vi "UHR-Fleezers Control (host) - Avogadro v2.vi"() -> ()   [LabVIEW 2014] (continued)
            }
            frame Enabled {
            }
          }
          "connection reference" <- w1502
          n930 = local write "connection reference"(w1502) -> ()
          n931 = local write "Database link"(w1501) -> ()
        }
        frame #3 {
          # "Load active calibration to fpga"
          n932 = local read "Base N trap periods"() -> (w1506:u32)
          n933 = local read "T1 Osc Enable"() -> (w1505:bool)
          n934 = property on="T1 Osc Enable" class="Bool (strict)"("Val(Sgnl)"=w1505) -> ()  [unwired: 2 in, 2 out]
          n935 = property on="Base N trap periods" class="DigNum (strict)"("Val(Sgnl)"=w1506) -> ()  [unwired: 2 in, 2 out]
        }
      }
    }
    frame #4 {
      # "Set FIFO size and run FPGA"
      n936 = local read "FPGA error out"() -> (w1508:errorcluster)
      n937 = xnode "Invoke Method"("FPGA VI Reference In"=w1509, "error in"=w1508, "Requested Depth"="Trap AI FIFO Depth") -> ("FPGA VI Reference Out"=w1513:T40, "error out"=w1514:errorcluster)  [unwired: 1 out]
      n938 = xnode "Invoke Method"("FPGA VI Reference In"=w1513, "error in"=w1514, "Requested Depth"="Trap Position FIFO Depth") -> ("FPGA VI Reference Out"=w1511:T40, "error out"=w1510:errorcluster)  [unwired: 1 out]
      n939 = xnode "Invoke Method"("FPGA VI Reference In"=w1511, "error in"=w1510) -> ("error out"=w1507:errorcluster)  [unwired: 1 in, 1 out]
      n940 = local write "FPGA error out"(w1507) -> ()
    }
    frame #5 {
      # "Adjust FPGA timing loop phases"
      n941 = flat-sequence "Initial FPGA Loop Relative Phase Adjustment" {
        tunnel: "Initial Phase Adjustment (AI1)" -> [w1548]
        tunnel: "Initial Phase Adjustment (GI)" -> [w1547]
        tunnel: "Initial Phase Adj. (MCL)" -> [w1546]
        tunnel: [w1549] -> w1533
        tunnel: [w1545] -> w1532
        tunnel: "Initial Phase Adjustment (APD Acq)" -> [w1544]
        tunnel: "Initial Phase Adjustment (APD 1 Gate)" -> [w1543]
        tunnel: "Initial Phase Adjustment (Green FB)" -> [w1542]
        tunnel: "Initial Phase Adjustment (GI) 2" -> [w1541]
        tunnel: "Initial Phase Adjustment (APD 2 Gate)" -> [w1540]
        tunnel: "Initial Phase Adjustment (RI)" -> [w1539]
        tunnel: "Initial Phase Adjustment (BI DO)" -> [w1538]
        tunnel: "Initial Phase Adjustment (BI AO)" -> [w1537]
        tunnel: "Initial Phase Adjustment (APD 3 Gate)" -> [w1536]
        tunnel: w1518 -> [w1535]
        tunnel: w1533 -> [w1551]
        tunnel: [w1552] -> w1531
        tunnel: w1532 -> [w1552]
        tunnel: [w1551] -> w1530
        tunnel: w1531 -> [w1556]
        tunnel: w1530 -> [w1555]
        tunnel: [w1553] -> w1517
        frame #0 {
          n942 = local read "FPGA error out"() -> (w1534:errorcluster)
          n943 = xnode "Read/Write Control"("FPGA VI Reference In"=w1535, "error in"=w1534, "Phase count adjustment"=w1548, "Phase count adjustment (GI)"=w1547, "Phase count adjustment (MCL)"=w1546, "Phase Count Adjustment (APD Acq)"=w1544, "Phase count adjustment (APD 1 Gate)"=w1543, "Phase count adjustment (APD 2 Gate)"=w1540, "Phase count adjustment (Green FB)"=w1542, "Phase count adjustment (GI) 2"=w1541, "Phase count adjustment (RI)"=w1539, "Phase count adjustment (BI AO)"=w1537, "Phase count adjustment (BI D)"=w1538, "Phase count adjustment (APD 3 Gate)"=w1536) -> ("FPGA VI Reference Out"=w1545:T40, "error out"=w1549:errorcluster)
        }
        frame #1 {
          n944 = Wait (ms)(milliseconds to wait=u32 100) -> ()  [unwired: 1 out]
        }
        frame #2 {
          w1554 = TRUE
          n945 = xnode "Read/Write Control"("FPGA VI Reference In"=w1556, "error in"=w1555, "+ phase"=w1554, "+ phase (GI)"=w1554, "+ phase (MCL)"=w1554, "+ phase (APD Acq)"=w1554, "+ phase (APD 1 Gate)"=w1554, "+ phase (APD 2 Gate)"=w1554, "+ phase (Green FB)"=w1554, "+ phase (GI) 2"=w1554, "+ phase (RI)"=w1554, "+ phase (BI AO)"=w1554, "+ phase (BI D)"=w1554, "+ phase (APD 3 Gate)"=w1554) -> ("error out"=w1553:errorcluster)  [unwired: 1 out]
        }
      }
      n946 = local write "FPGA error out"(w1517) -> ()
    }
    frame #6 {
      w1572 = 6.0  # clock mult.
      w1571 = 49152000.0  # TCXO frequ.
      w1576 = 6.0  # clock mult.
      w1577 = 49152000.0  # TCXO frequ.
      # "Added by ronen - definition of \nlimit frequencies when using dynamic feedback"
      # "Initialize trap RF synth board and set initial frequencies and amplitudes"
      n947 = local read "FPGA error out"() -> (w1557:errorcluster)
      n948 = call "set RF board frequency - interlace.vi"("Board 2 Frequency Limits"=w1583, "Board 1 Frequency Limits"=w1564, "error in"=w1557, "FPGA VI Reference In"=w1558, "Board 2 Frequency 3 (MHz)"="BD 2 Frequency 3 (MHz)", "Board 1 Frequency 3 (MHz)"="BD 1 Frequency 3 (MHz)", "Board 2 Frequency 2 (MHz)"="BD 2 Frequency 2 (MHz)", "Board 2 Frequency 1 (MHz)"="BD 2 Frequency 1 (MHz)", "Board 1 Frequency 2 (MHz)"="BD 1 Frequency 2 (MHz)", "Board 1 Frequency 1  (MHz)"="BD 1 Frequency 1 (MHz)") -> ("error out"=w1588:errorcluster, "FPGA VI Reference Out"=w1563:T40)
      n949 = Unbundle By Name(w1564) -> ("Maximum"=w1574:dbl, "Minimum"=w1565:dbl)
      n950 = call "set RF board amplitude - interlace.vi"("Board 2 Amplitude Limits"=w1585, "Board 1 Amplitude Limits"=w1584, "error in"=w1588, "FPGA VI Reference In"=w1563, "Board 2 Amplitude 3 (%)"="BD 2 Amplitude 3 (%)", "Board 1 Amplitude 3 (%)"="BD 1 Amplitude 3 (%)", "Board 2 Amplitude 2 (%)"="BD 2 Amplitude 2 (%)", "Board 2 Amplitude 1 (%)"="BD 2 Amplitude 1 (%)", "Board 1 Amplitude 2 (%)"="BD 1 Amplitude 2 (%)", "Board 1 Amplitude 1 (%)"="BD 1 Amplitude 1 (%)") -> ("error out"=w1560:errorcluster)  [unwired: 1 out]
      n951 = Multiply(x=w1565, y=1000000.0) -> (x*y=w1569:dbl)
      n952 = Multiply(x=w1574, y=1000000.0) -> (x*y=w1579:dbl)
      n953 = Scale By Power Of 2(n=48, x=w1569) -> (x*2^n=w1567:dbl)
      n954 = Subtract(x="BD 1 Frequency 1 (MHz)", y="BD 1 Frequency 2 (MHz)") -> (x-y=w1595:dbl)
      n955 = Subtract(x="BD 2 Frequency 1 (MHz)", y="BD 2 Frequency 2 (MHz)") -> (x-y=w1596:dbl)
      n956 = Scale By Power Of 2(n=48, x=w1579) -> (x*2^n=w1581:dbl)
      n957 = Multiply(x=w1571, y=w1572) -> (x*y=w1573:dbl)
      n958 = Multiply(x=w1577, y=w1576) -> (x*y=w1575:dbl)
      n959 = Square(x=w1596) -> (x^2=w1598:dbl)
      n960 = Square(x=w1595) -> (x^2=w1597:dbl)
      n961 = Divide(x=w1567, y=w1573) -> (x/y=w1568:dbl)
      n962 = Divide(x=w1581, y=w1575) -> (x/y=w1580:dbl)
      n963 = Add(x=w1597, y=w1598) -> (x+y=w1599:dbl)
      n964 = To Unsigned Quad Integer(1:w1568) -> (0:w1561:u64)
      n965 = To Unsigned Quad Integer(1:w1580) -> (0:w1562:u64)
      n966 = Square Root(x=w1599) -> (sqrt(x)=w1600:dbl)
      n967 = local write "Trap Delta (MHz)"(w1600) -> ()
      n968 = xnode "Read/Write Control"("FPGA VI Reference In"=w1563, "error in"=w1560, "FB Max Frequency"=w1562, "FB Min frequency"=w1561) -> ("error out"=w1559:errorcluster)  [unwired: 1 out]
      n969 = local write "FPGA error out"(w1559) -> ()
    }
    frame #7 {
      n970 = flat-sequence {
        frame #0 {
          n971 = local read "Trap 1 (ON/OFF)"() -> (w1605:bool)
          n972 = local write "Saving..."(FALSE ("Saving Data")) -> ()
          n973 = local write "Stop All"(FALSE ("Stop All")) -> ()
          n974 = local write "Index"(1.0 ("Index")) -> ()
          n975 = property on="Trap 1 ON" class="Bool (strict)"("Value"=w1605) -> ()  [unwired: 2 in, 2 out]
          "Manipulating Trap" <- FALSE ("Manipulating Trap")
        }
        frame #1 {
          n976 = local read "Trap 2 (ON/OFF)"() -> (w1610:bool)
          n977 = Wait (ms)(milliseconds to wait=u32 10) -> ()  [unwired: 1 out]
          n978 = property on="Trap 2 ON" class="Bool (strict)"("Val(Sgnl)"=w1610) -> ()  [unwired: 2 in, 2 out]
        }
        frame #2 {
          n979 = local read "Scan Range (nm)"() -> (w1612:dbl)
          n980 = call "Update messages.vi"("Message to add"="UHR-Fleezers ready.", "Old message string"="") -> ("New message string"=w1615:string)
          n981 = local write "Messages"(w1615) -> ()
          n982 = property on="Scan Range (nm)" class="DigNum (strict)"("Val(Sgnl)"=w1612) -> ()  [unwired: 2 in, 2 out]
        }
      }
    }
    frame #8 {
      w1646 = 0
      w1645 = 2
      w1644 = 0
      w1641 = 3
      w1640 = 2
      w1639 = 5
      w1637 = 1
      w1636 = 2
      w1678 = u32 0
      w1684 = cluster{u32, u32} {16777238, 16777238}
      w1679 = 0.0
      # "Initialize the multi-MCL offset array"
      # "Initialize valves"
      # "Cursor control of trap\n3"
      # "Graph of positions and displacements in 2D"
      n983 = local read "MCL offset scanning range (V)"() -> (w1665:T4)
      n984 = control-ref of="Positions \nand displacements"() -> (w1616:refnum<vi>)
      n985 = local read "Offset file step size"() -> (w1668:dbl)
      n986 = Divide(x=30.0, y=w1668) -> (x/y=w1659:dbl)
      n987 = call "start_stage_trackball.vi"("Enum"=T45."Trackball XY", "Stage Controller port"=w1672) -> ("error out"=w1670:errorcluster)  [unwired: 1 in, 1 out]
      n988 = Initialize Array(0.0, w1659) -> (w1666:dbl[])
      n989 = call "Make Trap3 position array.vi"("MCL offset scanning range (V)"=w1665) -> ("X Data points"=w1658:u64, "Y data points"=w1661:u64)  [unwired: 3 out]
      n990 = property on="Stage Control Serial Error" class="Clust (strict)"("Val(Sgnl)"=w1670) -> ()  [unwired: 2 in, 2 out]
      n991 = Bundle(w1666, w1666, w1666, w1666, w1666, w1666) -> (w1663:T50)  [unwired: 1 in]
      n992 = Multiply(x=w1661, y=w1658) -> (x*y=w1664:u64)
      n993 = for {
        N: w1664 -> [_]
        tunnel: [w1695] -> w1662 mode=indexing
        tunnel: w1663 -> [w1695]
      }
      n994 = Build Array("T1", "T2", "T3", "disp1", "disp2", "disp3", "junc1", "junc2", "junc3", "Mean Junc") -> (w1657:string[])
      n995 = property class="XYGraph (strict)"(reference=w1616, "Legend:Plots Shown"=10, "XScale.Maximum"=7900.0, "XScale.Minimum"=1000.0, "YScale.Maximum"=400.0, "YScale.Minimum"=-3200.0, "Frame Color"=u32 9868950) -> (reference out=w1624:refnum<vi>)  [unwired: 1 in, 1 out]
      n996 = Reshape Array(w1662, w1658, w1661) -> (w1660:T51)
      n997 = local write "Multi-MCL offset array"(w1660) -> ()
      n998 = Build Array(u32 16711680, u32 16711680, u32 16711680, u32 40779, u32 40779, u32 40779, u32 16711898, u32 16711898, u32 16711898, u32 16860) -> (w1635:u32[])
      n999 = Build Array(w1636, w1636, w1636, w1637, w1637, w1637, w1637, w1637, w1637, w1637) -> (w1638:i32[])
      n1000 = Build Array(w1639, w1639, w1639, w1640, w1640, w1640, w1641, w1641, w1641, 5) -> (w1643:i32[])
      n1001 = Build Array(w1644, w1644, w1644, w1645, w1645, w1645, w1646, w1646, w1646, w1646) -> (w1647:i32[])
      n1002 = for {
        tunnel: w1624 -> [w1694]
        tunnel: w1635 -> [w1692] mode=indexing
        tunnel: w1638 -> [w1691] mode=indexing
        tunnel: w1643 -> [w1690] mode=indexing
        tunnel: w1647 -> [w1689] mode=indexing
        tunnel: w1657 -> [w1687] mode=indexing
        i -> [w1693]
        n1003 = property class="XYGraph (strict)"(reference=w1694, "Active Plot"=w1693) -> (reference out=w1688:refnum<vi>)  [unwired: 1 in, 1 out]
        n1004 = property class="XYGraph (strict)"(reference=w1688, "Plot.Fill/Pt. Color"=w1692, "Plot.Point Style"=w1691, "Plot.Line Width"=w1690, "Plot.Plot Interpolation"=w1689, "Plot.Plot Name"=w1687) -> ()  [unwired: 1 in, 2 out]
      }
      n1005 = control-ref of="Piezo trap cursor control"() -> (w1680:refnum<vi>)
      n1006 = property class="XYGraph (strict)"(reference=w1680, "XScale.Maximum"=10.0, "XScale.Minimum"=w1679, "YScale.Maximum"=w1679, "YScale.Minimum"=-10.0, "Plot Area Colors"=w1684, "Frame Color"=u32 9868950, "XScale.GridColors"=w1684, "YScale.GridColors"=w1684, "Cursor.Cursor Color"=u32 16711680, "Active Cursor"=w1678, "Cursor.CursorMode"=w1678) -> ()  [unwired: 1 in, 2 out]
      n1007 = call "hamilton_controller.vi"("VISA resource name in"="Visa resource for valves", "action"=T48."CONNECT") -> ("error out"=w1677:errorcluster, "VISA resource name out"=w1674:refnum<visa-resource-name>)  [unwired: 8 in]
      n1008 = call "hamilton_controller.vi"("VISA resource name in"=w1674, "error in"=w1677, "action"=T48."INITIALIZE VALVES") -> ("error out"=w1686:errorcluster)  [unwired: 7 in, 1 out]
    }
    frame #9 {
      # "Wait 5 s for all the event loops still being executed to finish."
      n1009 = Wait (ms)(milliseconds to wait=u32 5000) -> ()  [unwired: 1 out]
      n1010 = local read "FPGA error out"() -> (w1697:errorcluster)
    }
  }
  n1011 = node-c288() -> (w31:T42)  [unwired: 4 out]
  n1012 = disable-structure shown="Disabled" {
    frame Disabled {
      n1013 = while "Duncan's play event loop" {
        stop <- w1701 stop-if-true
        n1014 = Create User Event(user event datatype=TRUE ("Boolean")) -> (user event=w1702:refnum<user-event>)  [unwired: 1 in, 1 out]
        n1015 = Create User Event(user event datatype=TRUE ("Boolean")) -> (user event=w1708:refnum<user-event>)  [unwired: 1 in, 1 out]
        n1016 = global write "Global for fluorescence simulation mean (30 samples), (power series).vi" "Red Signal"(w1702) -> ()
        n1017 = global write "Global for fluorescence simulation mean (30 samples), (power series).vi" "Green Signal"(w1708) -> ()
        n1018 = register-events(w1708, w1702) -> (reference out=w1707:refnum<event-registration>)  [unwired: 2 in, 1 out]
        n1019 = event shown="[1] \"Start assembly line\": Value Change" {
          selector: w1707 -> [_ _ _ _]
          dyn-events: _ -> [_ _ _ _]
          timeout: 100 -> [_ _ _ _]
          event Timeout {
            n1020 = event-data() -> ()  [unwired: 1 in, 2 out]
          }
          event "Start assembly line": Value Change {
            n1021 = event-data() -> ("OldVal"=w1710:bool)  [unwired: 1 in, 4 out]
            n1022 = case shown="True" w1710 {
              selector: w1710 -> [_ w1711]
              frame False {
              }
              frame True {
                n1023 = property on="Move to Position 3" class="Bool (strict)"("Val(Sgnl)"=w1711) -> ()  [unwired: 2 in, 2 out]
                n1024 = case shown="1" "Numeric" {
                  frame 0, Default {
                  }
                  frame 1 {
                    n1025 = property on="Green Laser ON" class="Bool (strict)"("Val(Sgnl)"=TRUE ("Value (Signaling)")) -> ()  [unwired: 2 in, 2 out]
                  }
                  frame 2 {
                    n1026 = property on="Red Laser ON" class="Bool (strict)"("Val(Sgnl)"=TRUE) -> ()  [unwired: 2 in, 2 out]
                  }
                }
              }
            }
          }
          event User Event {
            n1027 = event-data() -> ("Boolean"=w1715:bool)  [unwired: 1 in, 3 out]
            "Green Fluorophore" <- w1715
            n1028 = property on="Start assembly line" class="Bool"("Val(Sgnl)"=w1715) -> ()  [unwired: 2 in, 2 out]
          }
          event User Event {
            n1029 = event-data() -> ("Boolean"=w1716:bool)  [unwired: 1 in, 3 out]
            "Red Fluorophore" <- w1716
            n1030 = property on="Start assembly line" class="Bool"("Val(Sgnl)"=w1716) -> ()  [unwired: 2 in, 2 out]
          }
        }
        n1031 = property on="Get Fluorophore" class="Bool (strict)"("Val(Sgnl)"="Get Fluorophore") -> ()  [unwired: 2 in, 2 out]
        n1032 = Wait (ms)(milliseconds to wait=u32 100) -> ()  [unwired: 1 out]
        n1033 = local read "Stop All"() -> (w1700:bool)
        n1034 = Or(x=w1700, y="stop") -> (x .or. y?=w1701:bool)
      }
    }
    frame Enabled {
    }
  }
  n1035 = timed-loop "Rough control of MCL mirror stage (debugging)" {
    tunnel: [w1719] -> w71
    timing: w31 -> [_]
    timing-out: [_] -> w30
    tunnel: w26 -> [w1717]
    stop <- w1719 stop-if-true
    n1036 = node-c288() -> ()  [unwired: 2 out]
    n1037 = case shown="1" "MCL Mode" {
      tunnel: w1717 -> [_ w1722 w1769]
      frame 0, Default {
      }
      frame 1 {
        n1038 = node-c288() -> (w1724:T42)  [unwired: 4 out]
        n1039 = timed-loop "Oscillate MCL mirror" {
          timing: w1724 -> [_]
          timing-out: [_] -> w1723
          tunnel: w1722 -> [w1725]
          i -> [w1763]
          stop <- w1726 stop-if-true
          n1040 = node-c288() -> (w1762:i64)  [unwired: 1 out]
          n1041 = Multiply(x="AO1", y=32767.0) -> (x*y=w1758:dbl)
          n1042 = Multiply(x="AO2", y=32767.0) -> (x*y=w1753:dbl)
          n1043 = Divide(x=w1758, y=10.0) -> (x/y=w1759:dbl)
          n1044 = Divide(x=w1753, y=10.0) -> (x/y=w1754:dbl)
          n1045 = To Word Integer(number=w1759) -> (16bit integer=w1751:i16)
          n1046 = To Word Integer(number=w1754) -> (16bit integer=w1750:i16)
          n1047 = Divide(x=w1762, y=i64 1000) -> (x/y=w1733:dbl)
          n1048 = Multiply(x=w1733, y=w1763) -> (x*y=w1744:dbl)
          n1049 = Multiply(x="Osc. freq. (Hz) 2", y=6.283185307179586) -> (x*y=w1745:dbl)
          n1050 = Multiply(x=w1745, y=w1744) -> (x*y=w1743:dbl)
          n1051 = Sine(x=w1743) -> (sin(x)=w1742:dbl)
          n1052 = Multiply(x=w1742, y="Osc. amp. (V)") -> (x*y=w1740:dbl)
          n1053 = Add(x=w1740, y="Osc. center (V)") -> (x+y=w1738:dbl)
          n1054 = Divide(x=w1738, y=10.0) -> (x/y=w1736:dbl)
          n1055 = Multiply(x=w1736, y=32767.0) -> (x*y=w1731:dbl)
          n1056 = Select(t=w1731, s="Scan axis", f=w1751) -> (s? t:f=w1749:dbl)
          n1057 = Select(t=w1750, s="Scan axis", f=w1731) -> (s? t:f=w1748:dbl)
          n1058 = local read "MCL Mode"() -> (w1730:u16)
          n1059 = Not Equal?(x=w1730, y=u16 1) -> (x != y?=w1727:bool)
          n1060 = local read "Stop All"() -> (w1728:bool)
          n1061 = xnode "Read/Write Control"("FPGA VI Reference In"=w1725, "AO1 (Y)"=w1749, "AO2 (X)"=w1748) -> ()  [unwired: 1 in, 2 out]
          n1062 = Compound Arithmetic op=OR(w1728, w1727) -> (w1726:bool)
          n1063 = node-c288() -> ()  [unwired: 2 out]
        }
        n1064 = node-c288(w1723) -> ()  [unwired: 1 out]
      }
      frame 2 {
        n1065 = case shown="True" "Start Scan" {
          tunnel: w1769 -> [_ w1771]
          frame False {
          }
          frame True {
            n1066 = Subtract(x="End (V)", y="Begin (V)") -> (x-y=w1778:dbl)
            n1067 = Decrement(x="N Points") -> (x-1=w1777:dbl)
            n1068 = Divide(x=w1778, y=w1777) -> (x/y=w1775:dbl)
            n1069 = for {
              N: "N Points" -> [_]
              tunnel: "Begin (V)" -> [w1794]
              tunnel: [w1786] -> w1781 mode=indexing
              tunnel: w1775 -> [w1785]
              tunnel: [w1783] -> w1774 mode=indexing
              tunnel: w1771 -> [w1782]
              i -> [w1793]
              n1070 = Multiply(x=w1785, y=w1793) -> (x*y=w1792:dbl)
              n1071 = Add(x=w1794, y=w1792) -> (x+y=w1789:dbl)
              n1072 = local read "Scan axis"() -> (w1784:bool)
              n1073 = local read "AO1"() -> (w1791:dbl)
              n1074 = local read "AO2"() -> (w1790:dbl)
              n1075 = Select(t=w1789, s=w1784, f=w1791) -> (s? t:f=w1788:dbl)
              n1076 = Select(t=w1790, s=w1784, f=w1789) -> (s? t:f=w1787:dbl)
              n1077 = flat-sequence {
                tunnel: w1788 -> [w1798]
                tunnel: w1787 -> [w1797]
                tunnel: w1782 -> [w1795]
                tunnel: [w1808] -> w1786
                tunnel: [w1807] -> w1783
                frame #0 {
                  w1801 = 10.0 ("y")
                  w1796 = 32767.0 ("y")
                  n1078 = Multiply(x=w1798, y=w1796) -> (x*y=w1804:dbl)
                  n1079 = Multiply(x=w1797, y=w1796) -> (x*y=w1802:dbl)
                  n1080 = Divide(x=w1804, y=w1801) -> (x/y=w1805:dbl)
                  n1081 = Divide(x=w1802, y=w1801) -> (x/y=w1803:dbl)
                  n1082 = To Word Integer(number=w1805) -> (16bit integer=w1799:i16)
                  n1083 = To Word Integer(number=w1803) -> (16bit integer=w1800:i16)
                  n1084 = xnode "Read/Write Control"("FPGA VI Reference In"=w1795, "AO1 (Y)"=w1799, "AO2 (X)"=w1800) -> ()  [unwired: 1 in, 2 out]
                }
                frame #1 {
                  n1085 = Wait (ms)(milliseconds to wait="DAQ Delay (ms)") -> ()  [unwired: 1 out]
                }
                frame #2 {
                  n1086 = local read "Slow mean"() -> (w1808:dbl)
                  n1087 = local read "Sigma"() -> (w1807:dbl)
                }
              }
            }
            n1088 = Bundle("Begin (V)"="Begin (V)", w1775, w1781) -> (→"MCL Scan":cluster{"Begin (V)":dbl, dbl, dbl[]})  [unwired: 1 out]
            n1089 = Bundle("Begin (V)"="Begin (V)", w1775, w1774) -> (→"MCL Scan 2":cluster{"Begin (V)":dbl, dbl, dbl[]})  [unwired: 1 out]
          }
        }
      }
    }
    n1090 = local read "Stop All"() -> (w1719:bool)
    n1091 = node-c288() -> ()  [unwired: 2 out]
  }
  n1092 = node-c288(w30) -> ()  [unwired: 1 out]
  n1093 = node-c288(2 ("Processor")) -> (w62:T42)  [unwired: 3 out]
  n1094 = timed-loop "Basic control parameters (all FPGA settings, other basic controls)" {
    shift-right: [w1816] -> _
    shift-left: errorcluster {"status"=FALSE, "code"=0, "source"=""} ("error out") -> [_]
    tunnel: [w1815] -> _
    timing: w62 -> [_]
    timing-out: [_] -> w61
    tunnel: w44 -> [w1814]
    tunnel: w40 -> [w1813]
    tunnel: w39 -> [w1812]
    tunnel: w38 -> [w1811]
    tunnel: w37 -> [w1810]
    tunnel: w26 -> [w1809]
    stop <- w1815 stop-if-true
    n1095 = node-c288() -> ()  [unwired: 2 out]
    n1096 = event shown="[27] \"Invert APD Gate\", \"APD Gate ON Count\", \"APD Gate OFF Count\", \"APD Gate\", \"APD Integration Time (s)\", \"APD AO Scale Factor\", \"Duty Frequency (ON 1/N cycles)\", \"Interlace ON count\", \"Interlace OFF count\": Value Change" {
      selector: _ -> [_ _ _ _ _ _ _ _ _ _ _ _ _ _ _ _ _ _ _ _ _ _ _ _ _ _ _ _ _ _ _ _ _ _ _ _ _ _ _ _ _ _ _ _ _ _ _ _ _ _ _ _ _ _ _ _ _ _ _ _ _ _ _ _ _ _ _ _ _ _ _ _ _ _ _ _ _ _ _ _ _ _ _ _ _ _ _ _ _ _ _ _]
      dyn-events: _ -> [_ _ _ _ _ _ _ _ _ _ _ _ _ _ _ _ _ _ _ _ _ _ _ _ _ _ _ _ _ _ _ _ _ _ _ _ _ _ _ _ _ _ _ _ _ _ _ _ _ _ _ _ _ _ _ _ _ _ _ _ _ _ _ _ _ _ _ _ _ _ _ _ _ _ _ _ _ _ _ _ _ _ _ _ _ _ _ _ _ _ _ _]
      timeout: _ -> [_ _ _ _ _ _ _ _ _ _ _ _ _ _ _ _ _ _ _ _ _ _ _ _ _ _ _ _ _ _ _ _ _ _ _ _ _ _ _ _ _ _ _ _ _ _ _ _ _ _ _ _ _ _ _ _ _ _ _ _ _ _ _ _ _ _ _ _ _ _ _ _ _ _ _ _ _ _ _ _ _ _ _ _ _ _ _ _ _ _ _ _]
      tunnel: [w1856 _ _ _ w1883 _ _ _ _ _ _ _ w1989 _ _ w2080 w2082 w2089 w2091 w2161 _ w2203 w2230 w2258 w2283 w2310 w2336 w2365 _ w2370 w2464 w2468 w2505 _ w2598 w2601 w2604 w2614 w2617 _ w2624 _ _ _ _ _ _ _ _ _ _ _ _ _ _ _ _ _ _ _ w3169 _ _ _ _ w3206 _ _ _ _ _ _ _ _ _ _ _ _ _ _ _ _ _ _ _ _ _ _ _ _ _ _] -> w1816
      tunnel: [_ _ _ _ _ _ _ _ _ _ w1968 _ _ _ _ _ _ _ _ _ _ _ _ _ _ _ _ _ _ _ _ _ _ _ _ _ _ _ _ _ _ _ _ _ _ _ _ _ _ _ _ _ _ _ _ _ _ _ _ _ _ _ _ _ _ _ _ _ _ _ _ _ _ _ _ _ _ _ _ _ _ _ _ _ _ _ _ _ _ _ _ _] -> w1815
      tunnel: [_ _ _ _ _ _ _ _ "Round T1 X" _ _ _ _ _ _ _ _ _ _ _ _ _ _ _ _ _ _ _ _ _ _ _ _ _ _ _ _ _ _ _ _ _ _ _ _ _ _ _ _ _ _ _ _ _ _ _ _ _ _ _ _ _ _ _ _ _ _ _ _ _ _ _ _ _ _ _ _ _ _ _ _ _ _ _ _ _ _ _ _ _ _ _] -> _
      tunnel: [_ _ _ "Adjust Scale\nto Mean" _ _ _ _ _ _ _ _ _ _ _ _ _ _ _ _ _ _ _ _ _ _ _ _ _ "Test ttrig" _ _ _ _ _ _ _ _ _ _ _ _ _ _ _ _ _ _ _ _ w2916 w2980 w3027 w3076 _ _ _ _ _ _ _ _ _ _ _ _ _ _ _ _ _ _ _ _ _ _ _ _ _ _ _ _ _ _ _ _ _ _ _ _ _ _] -> _
      tunnel: [_ _ _ _ _ _ _ _ _ "Round T2 X" _ "Delayed Interlace Start" _ _ _ _ _ _ _ _ _ _ _ _ _ _ _ _ _ _ _ _ _ _ _ _ _ _ _ _ _ _ _ _ _ _ _ _ _ _ _ _ _ _ _ _ _ _ _ _ _ _ _ _ _ _ _ _ _ _ _ _ _ _ _ _ _ _ _ _ _ _ _ _ _ _ _ _ _ _ _ _] -> _
      tunnel: w1814 -> [_ _ _ _ _ _ _ _ _ _ _ _ _ _ _ _ _ _ _ _ _ _ _ _ _ _ _ _ _ _ _ _ _ _ _ _ _ _ _ _ _ _ _ _ _ _ w2886 w2894 w2901 w2907 w2915 _ _ w3075 _ _ _ _ _ _ _ _ _ _ _ _ _ _ _ _ _ _ _ _ _ _ _ _ _ _ _ _ _ _ _ _ _ _ _ _ _ _]
      tunnel: w1813 -> [_ _ _ _ _ _ _ _ _ _ _ _ _ _ _ _ _ _ _ _ _ _ _ _ _ _ _ _ _ _ _ _ _ _ _ _ _ _ _ _ _ _ _ _ w2773 _ _ _ _ _ _ w2979 _ _ w3082 _ w3094 _ w3110 _ _ _ _ _ _ _ _ _ _ _ _ _ _ _ _ _ _ _ _ _ _ _ _ _ _ _ _ _ _ _ _ _]
      tunnel: w1812 -> [_ _ _ _ _ _ _ _ _ _ _ _ _ _ _ _ _ _ _ _ _ _ _ _ _ _ _ _ _ _ _ _ _ _ _ _ _ _ _ _ _ _ _ _ _ _ _ _ _ _ _ _ _ _ _ _ _ _ _ _ _ _ _ _ _ _ _ _ _ _ _ _ _ _ _ _ _ _ _ _ _ _ _ _ _ _ _ _ _ _ _ _]
      tunnel: w1811 -> [_ _ _ _ _ _ _ _ _ _ _ _ _ _ _ _ _ _ _ _ _ _ _ _ _ _ _ _ _ _ _ _ _ _ _ _ _ _ _ _ _ w2635 _ _ _ _ _ _ _ _ _ _ w3026 _ _ w3088 _ w3102 _ w3136 _ _ _ _ _ _ _ _ _ _ _ _ _ _ _ _ _ _ _ _ _ _ _ _ _ _ _ _ _ _ _ _]
      tunnel: w1810 -> [_ _ _ _ _ _ _ _ _ _ _ _ _ _ _ _ _ _ _ _ _ _ _ _ _ _ _ _ _ _ _ _ _ _ _ _ _ _ _ _ _ _ _ _ _ _ _ _ _ _ _ _ _ _ _ _ _ _ _ _ _ _ _ _ _ _ _ _ _ _ _ _ _ _ _ _ _ _ _ _ _ _ _ _ _ _ _ _ _ _ _ _]
      tunnel: w1809 -> [w1819 _ _ _ w1882 _ w1908 _ _ _ _ _ w1980 _ _ w2064 w2081 w2088 w2090 w2126 _ w2192 w2228 w2240 w2265 w2293 w2313 w2341 w2366 w2368 w2372 w2465 w2469 _ w2595 w2599 w2602 w2612 w2615 _ w2623 _ _ w2718 _ _ _ _ _ _ _ _ _ _ _ _ _ _ _ _ w3162 _ w3183 _ w3190 w3205 _ w3212 w3239 w3246 w3262 w3270 _ w3281 _ w3325 _ _ w3379 w3410 w3414 w3422 _ w3486 w3496 w3515 _ _ _ _ _ _]
      tunnel: [_ _ _ _ _ _ _ _ _ _ w1967 _ _ _ _ _ _ _ _ _ _ _ _ _ _ _ _ _ _ _ _ _ _ _ _ _ _ _ _ _ _ _ w2715 w2720 _ _ _ _ _ _ _ _ _ _ _ _ _ _ _ _ _ _ _ _ _ _ _ _ _ _ _ _ _ _ _ _ _ _ _ _ _ _ _ _ _ _ _ _ _ _ _ _] -> _
      event "AI Count (ticks)", "Sets to FIFO (Traps)", "Save ave N", "FPGA Ave.", "# Samples/channel", "N sets to save": Value Change {
        # "RG 18-01-16 Increased amount of elements to read for trap position, to add x and y for piezo trap"
        # "So that if 'Save ave N' is updated, the AOD scanning code updates too."
        n1097 = event-data() -> ()  [unwired: 6 out]
        n1098 = local read "AI Count (ticks)"() -> (w1840:u16)
        n1099 = Divide(x=40000000.0, y=w1840) -> (x/y=w1832:dbl)
        "AI rate (Hz)" <- w1832
        "Ave. Rate (Hz)" <- w1832
        n1100 = Reciprocal(x=w1832) -> (1/x=→"Ave. Period (s)":dbl)
        n1101 = Unbundle By Name("Sets to FIFO (Traps)") -> ("Set 1"=w1823:bool, "Set 2"=w1822:bool, "Set 3"=w1821:bool)
        n1102 = Divide(x=w1832, y="N Acq Sets (Traps + Fl.)") -> (x/y=w1853:dbl)
        "Data Rate (Hz)" <- w1853
        n1103 = Reciprocal(x=w1853) -> (1/x=→"Data Period (s)":dbl)
        n1104 = Boolean To (0,1)(Boolean="Sets to FIFO (Traps)") -> (0, 1=w1848:cluster{"Set 1":i16, "Set 2":i16, "Set 3":i16})
        n1105 = xnode "Read/Write Control"("FPGA VI Reference In"=w1819, "ai count"=w1840, "Set 1"=w1823, "Set 2"=w1822, "Set 3"=w1821, "N of AI1 Int Acq Sets"="N Acq Sets (Traps + Fl.)") -> ("error out"=w1856:errorcluster)  [unwired: 1 in, 1 out]
        n1106 = Cluster To Array(cluster=w1848) -> (array=w1847:i16[])
        n1107 = local read "Save ave N"() -> (w1852:dbl)
        n1108 = To Unsigned Long Integer(number=w1847) -> (unsigned 32bit integer=w1829:u32[])
        n1109 = local read "Scan steps (AOD)"() -> (w1849:u64)
        n1110 = Multiply(x=w1840, y="N Acq Sets (Traps + Fl.)") -> (x*y=w1838:u16)
        n1111 = Add Array Elements(numeric array=w1829) -> (sum=w1841:u32)
        "Trap Sets" <- w1841
        n1112 = Divide(x=w1853, y=w1852) -> (x/y=w1851:dbl)
        "Save Data Rate (Hz)" <- w1851
        n1113 = Reciprocal(x=w1851) -> (1/x=→"Save Data Period (s)":dbl)
        n1114 = property on="Scan steps (AOD)" class="DigNum (strict)"("Val(Sgnl)"=w1849) -> ()  [unwired: 2 in, 2 out]
        n1115 = Multiply(x=w1838, y="# Samples/trap") -> (x*y=w1836:u32)
        "Counts/DMA" <- w1836
        n1116 = property on="Trap Disp. Downsample" class="DigNum (strict)"("Maximum"="# Samples/trap") -> ()  [unwired: 2 in, 2 out]
        n1117 = Multiply(x=w1841, y="# Samples/trap") -> (x*y=w1830:u32)
        "# Samples/channel" <- w1830
        n1118 = Multiply(x=w1830, y=u32 8) -> (x*y=→"Trap AI Elements/DMA read":u32)
        n1119 = local read "APD Int. Count"() -> (w1837:u32)
        n1120 = Multiply(x=w1830, y=u32 5) -> (x*y=→"Trap Pos Elements/DMA read":u32)
        n1121 = Divide(x=w1836, y=w1837) -> (x/y=w1827:dbl)
        "APD Samples/FIFO Acq." <- w1827
        n1122 = Divide(x=w1836, y=40000000.0) -> (x/y=w1834:dbl)
        "DMA Update Period (s)" <- w1834
        n1123 = local read "Number of APDs"() -> (w1820:u8)
        n1124 = Multiply(x=w1820, y=w1827) -> (x*y=→"APD Elements/DMA read":dbl)
        n1125 = property on="APD Disp. Downsample" class="DigNum (strict)"("Maximum"=w1827) -> ()  [unwired: 2 in, 2 out]
        n1126 = local read "N sets to save"() -> (w1846:u32)
        n1127 = Multiply(x=w1834, y=w1846) -> (x*y=→"Total Time (s) 2":dbl)
        "FPGA Averaging" <- FALSE ("FPGA Averaging")
      }
      event "Remove Offset": Value Change {
        n1128 = event-data() -> ()  [unwired: 7 out]
        n1129 = local write "Remove Offset"(FALSE ("Remove Offset")) -> ()
        n1130 = local read "Bead Mean (nm)"() -> (w1858:dbl)
        n1131 = local read "Offset (nm)"() -> (w1859:dbl)
        n1132 = Add(x=w1858, y=w1859) -> (x+y=w1857:dbl)
        n1133 = local write "Offset (nm)"(w1857) -> ()
      }
      event "Detector Type": Value Change {
        n1134 = event-data() -> ()  [unwired: 7 out]
        n1135 = local read "AI labels"() -> (w1863:string[])
        n1136 = property on="High Res. Display" class="Ring (strict)"("Strings []"=w1863) -> ()  [unwired: 2 in, 2 out]
        n1137 = Build Array (concatenate)(w1863, "none") -> (w1864:string[])
        n1138 = property on="FFT 1 Choice 1" class="Ring (strict)"("Strings []"=w1864) -> ()  [unwired: 2 in, 2 out]
        n1139 = property on="FFT 1 Choice 2" class="Ring (strict)"("Strings []"=w1864) -> ()  [unwired: 2 in, 2 out]
        n1140 = property on="FFT 2 Choice 1" class="Ring (strict)"("Strings []"=w1864) -> ()  [unwired: 2 in, 2 out]
        n1141 = property on="FFT 2 Choice 2" class="Ring (strict)"("Strings []"=w1864) -> ()  [unwired: 2 in, 2 out]
        n1142 = Bundle("APD 1", "APD 2", "APD 3") -> (w1867:cluster{string, string, string})  [unwired: 1 out]
        n1143 = Cluster To Array(cluster=w1867) -> (array=w1865:string[])
        n1144 = Build Array (concatenate)(w1865, w1864) -> (w1869:string[])
        n1145 = Array Size(array=w1869) -> (size(s)=w1861:i32)
        n1146 = property on="Signals to Plot" class="LstBox (strict)"("Item Names"=w1869) -> ()  [unwired: 2 in, 2 out]
        n1147 = property on="Signals to Plot" class="LstBox (strict)"("Number of Rows"=w1861) -> ()  [unwired: 2 in, 2 out]
        n1148 = property on="All Signals" class="WFChart (strict)"("LegNumRows"=w1861) -> ()  [unwired: 2 in, 2 out]
      }
      event "Adjust Scale\nto Mean": Value Change {
        n1149 = event-data() -> ()  [unwired: 7 out]
        n1150 = local read "APD rates cluster"() -> (w1872:T2)
        n1151 = Unbundle By Name(w1872) -> ("APD 1 Rate (Hz)"=w1871:dbl)
        n1152 = Multiply(x=1000.0, y="Above (kHz)") -> (x*y=w1878:dbl)
        n1153 = Multiply(x=1000.0, y="Below (kHz)") -> (x*y=w1876:dbl)
        n1154 = Add(x=w1878, y=w1871) -> (x+y=w1873:dbl)
        n1155 = Subtract(x=w1871, y=w1876) -> (x-y=w1874:dbl)
        n1156 = property on="APD Chart" class="WFChart (strict)"("YScale.Minimum"=w1874) -> ()  [unwired: 2 in, 2 out]
        n1157 = property on="APD Chart" class="WFChart (strict)"("YScale.Maximum"=w1873) -> ()  [unwired: 2 in, 2 out]
      }
      event "Phase adj. (AI1)", "+ phase (AI1)", "- phase (AI1)": Value Change {
        n1158 = event-data() -> ()  [unwired: 7 out]
        n1159 = Negate(x="Phase adj. (AI1)") -> (-x=w1890:i16)
        n1160 = Select(t=w1890, s="- phase (AI1)", f="Phase adj. (AI1)") -> (s? t:f=w1889:i16)
        n1161 = xnode "Read/Write Control"("FPGA VI Reference In"=w1882, "Phase count adjustment"=w1889) -> ("FPGA VI Reference Out"=w1888:T40, "error out"=w1887:errorcluster)  [unwired: 2 in]
        n1162 = Or(x="- phase (AI1)", y="+ phase (AI1)") -> (x .or. y?=w1884:bool)
        n1163 = xnode "Read/Write Control"("FPGA VI Reference In"=w1888, "error in"=w1887, "+ phase"=w1884) -> ("error out"=w1883:errorcluster)  [unwired: 1 in, 1 out]
      }
      event "Signals to Plot": Double Click {
        w1902 = u32 9868950 ("Color Box")
        n1164 = event-data() -> ("Row"=w1893:i32)  [unwired: 9 out]
        n1165 = property on="All Signals" class="WFChart (strict)"("Active Plot"=w1893) -> (error out=w1892:errorcluster)  [unwired: 2 in, 1 out]
        n1166 = property on="All Signals" class="WFChart (strict)" props=["Plot", "Plot Color", "Plot", "Visible?"](error in=w1892) -> (error out=w1895:errorcluster, "Plot.Visible?"=w1894:bool)  [unwired: 1 in, 2 out]
        n1167 = Select(t=FALSE ("Plot.Visible"), s=w1894, f=TRUE ("Plot.Visible")) -> (s? t:f=w1897:bool)
        n1168 = property on="All Signals" class="WFChart (strict)"(error in=w1895, "Plot.Visible?"=w1897) -> (error out=w1896:errorcluster)  [unwired: 1 in, 1 out]
        n1169 = property on="All Signals" class="WFChart (strict)"(error in=w1896) -> (error out=w1898:errorcluster, "Plot.Plot Color"=w1899:u32)  [unwired: 1 in, 1 out]
        n1170 = property on="Signals to Plot" class="LstBox (strict)"(error in=w1898, "Active Row"=w1893) -> (error out=w1903:errorcluster)  [unwired: 1 in, 1 out]
        n1171 = Select(t=w1899, s=w1897, f=u32 0) -> (s? t:f=w1904:u32)
        n1172 = property on="Signals to Plot" class="LstBox (strict)"(error in=w1903, "CellFontColor"=w1904, "SelColor"=w1902, "CellBG"=w1902, "CellFontSize"=u32 20 ("Active Row:Cell Font:Size"), "CellFontBold"=TRUE ("Active Row:Cell Font:Bold")) -> ()  [unwired: 1 in, 2 out]
      }
      event "BD 1 Frequency 1 (MHz)", "BD 1 Frequency 2 (MHz)", "BD 1 Frequency 3 (MHz)", "BD 2 Frequency 1 (MHz)", "BD 2 Frequency 2 (MHz)", "BD 2 Frequency 3 (MHz)", "Trap Delta (MHz)", "Update all trap values": Value Change {
        # "This is so you can set trap frequencies\nvia local variables and then update\nall at once"
        n1173 = event-data() -> ("CtlRef"=w1912:refnum<vi>)  [unwired: 6 out]
        n1174 = control-ref of="Trap Delta (MHz)"() -> (w1911:refnum<vi>)
        n1175 = Equal?(x=w1911, y=w1912) -> (x = y?=w1910:bool)
        n1176 = local write "Update all trap values"(FALSE ("Update all trap values")) -> ()
        n1177 = case shown="False" "Oscillate Set 1" {
          tunnel: w1910 -> [w1926 _]
          tunnel: w1908 -> [w1924 _]
          frame False {
            n1178 = local read "BD 1 Frequency 2 (MHz)"() -> (w1922:dbl)
            n1179 = case shown="False" "Symmetric?" {
              tunnel: "Trap Delta (MHz)" -> [w1948 w1955]
              tunnel: [w1949 w1953] -> w1914
              tunnel: [w1947 w1950] -> w1916
              tunnel: w1922 -> [w1949 _]
              frame False {
                n1180 = Subtract(x=w1949, y=w1948) -> (x-y=w1947:dbl)
              }
              frame True {
                w1952 = 75
                n1181 = Divide(x=w1955, y=2.0) -> (x/y=w1951:dbl)
                n1182 = Add(x=w1951, y=w1952) -> (x+y=w1953:dbl)
                n1183 = Subtract(x=w1952, y=w1951) -> (x-y=w1950:dbl)
              }
            }
            n1184 = local read "BD 1 Frequency 1 (MHz)"() -> (w1917:dbl)
            n1185 = Not(x="Symmetric?") -> (.not. x?=w1920:bool)
            n1186 = And(x=w1920, y="move Con X?") -> (x .and. y?=w1918:bool)
            n1187 = Subtract(x=w1917, y=w1916) -> (x-y=w1915:dbl)
            n1188 = Select(t=w1916, s=w1926, f=w1917) -> (s? t:f=w1925:dbl)
            n1189 = local read "Y RF Frequency Limits (MHz)"() -> (w1927:T26)
            n1190 = case shown="True" w1918 {
              tunnel: w1915 -> [_ w1946]
              frame False {
              }
              frame True {
                n1191 = property on="AOM X Cal (nm/MHz)" class="DigNum (strict)"() -> ("Value"=w1945:dbl)  [unwired: 2 in, 2 out]
                n1192 = property on="MCL Step Position Ratio" class="DigNum (strict)"() -> ("Value"=w1939:dbl)  [unwired: 2 in, 2 out]
                n1193 = Compound Arithmetic op=MULTIPLY(w1946, w1945, w1939) -> (w1944:dbl)
                n1194 = property on="MCL X Cal (nm/V)" class="DigNum (strict)"() -> ("Value"=w1943:dbl)  [unwired: 2 in, 2 out]
                n1195 = Divide(x=w1944, y=w1943) -> (x/y=w1942:dbl)
                n1196 = property on="AO2" class="Slide (strict)"() -> ("Value"=w1941:dbl)  [unwired: 2 in, 2 out]
                n1197 = Add(x=w1942, y=w1941) -> (x+y=w1940:dbl)
                n1198 = property on="AO2" class="Slide (strict)"("Val(Sgnl)"=w1940) -> ()  [unwired: 2 in, 2 out]
              }
            }
            n1199 = local read "X RF Frequency Limits (MHz)"() -> (w1928:T26)
            n1200 = local write "BD 1 Frequency 1 (MHz)"(w1925) -> ()
            n1201 = local read "BD 1 Frequency 3 (MHz)"() -> (w1937:dbl)
            n1202 = local read "BD 2 Frequency 1 (MHz)"() -> (w1931:dbl)
            n1203 = local read "BD 2 Frequency 2 (MHz)"() -> (w1930:dbl)
            n1204 = local read "BD 2 Frequency 3 (MHz)"() -> (w1938:dbl)
            n1205 = call "set RF board frequency - interlace.vi"("Board 2 Frequency Limits"=w1927, "Board 1 Frequency Limits"=w1928, "FPGA VI Reference In"=w1924, "Board 2 Frequency 3 (MHz)"=w1938, "Board 1 Frequency 3 (MHz)"=w1937, "Board 2 Frequency 2 (MHz)"=w1930, "Board 2 Frequency 1 (MHz)"=w1931, "Board 1 Frequency 2 (MHz)"=w1914, "Board 1 Frequency 1  (MHz)"=w1925) -> ()  [unwired: 1 in, 2 out]
            n1206 = Subtract(x=w1931, y=w1930) -> (x-y=w1935:dbl)
            n1207 = local write "BD 1 Frequency 2 (MHz)"(w1914) -> ()
            n1208 = Subtract(x=w1925, y=w1914) -> (x-y=w1936:dbl)
            n1209 = Square(x=w1935) -> (x^2=w1933:dbl)
            n1210 = Square(x=w1936) -> (x^2=w1934:dbl)
            n1211 = Add(x=w1934, y=w1933) -> (x+y=w1932:dbl)
            n1212 = Square Root(x=w1932) -> (sqrt(x)=w1929:dbl)
            n1213 = property on="Initial delta (MHz)" class="DigNum (strict)"("Val(Sgnl)"=w1929) -> ()  [unwired: 2 in, 2 out]
            n1214 = local write "Trap Delta (MHz)"(w1929) -> ()
          }
          frame True {
          }
        }
      }
      event "manual raster set": Value Change {
        n1215 = event-data() -> ()  [unwired: 7 out]
        n1216 = flat-sequence {
          frame #0 {
            n1217 = Replace Array Subset(array=u32[] [0] ("Index Values"), new element="manual raster set", index=0) -> (w1956:u32[])
            n1218 = property on="Saved AOD Raster Scan Parameter Sets" class="Arr (strict)"("Index Values"=w1956) -> ()  [unwired: 2 in, 2 out]
          }
          frame #1 {
            n1219 = property on="Load parameters" class="Bool (strict)"("Val(Sgnl)"=TRUE ("Value (Signaling)")) -> ()  [unwired: 2 in, 2 out]
          }
        }
      }
      event "Round T1 X": Value Change {
        n1220 = event-data() -> ()  [unwired: 7 out]
        n1221 = local read "BD 1 Frequency 1 (MHz)"() -> (w1963:dbl)
        n1222 = Round To Nearest(number=w1963) -> (nearest integer value=w1962:dbl)
        n1223 = property on="BD 1 Frequency 1 (MHz)" class="DigNum (strict)"("Val(Sgnl)"=w1962) -> ()  [unwired: 2 in, 2 out]
      }
      event "Round T2 X": Value Change {
        n1224 = event-data() -> ()  [unwired: 7 out]
        n1225 = local read "BD 1 Frequency 2 (MHz)"() -> (w1965:dbl)
        n1226 = Round To Nearest(number=w1965) -> (nearest integer value=w1964:dbl)
        n1227 = property on="BD 1 Frequency 2 (MHz)" class="DigNum (strict)"("Val(Sgnl)"=w1964) -> ()  [unwired: 2 in, 2 out]
      }
      event "Stop All": Value Change {
        n1228 = event-data() -> ()  [unwired: 7 out]
        n1229 = flat-sequence {
          tunnel: [w1971] -> w1969
          tunnel: [w1974] -> w1967
          tunnel: w1969 -> [w1974]
          tunnel: [TRUE] -> w1968
          frame #0 {
            n1230 = local read "Visa resource for valves"() -> (w1970:refnum<visa-resource-name>)
            n1231 = call "hamilton_controller.vi"("VISA resource name in"=w1970, "action"=T48."DISCONNECT") -> ("error out"=w1971:errorcluster)  [unwired: 8 in, 1 out]
          }
          frame #1 {
          }
        }
      }
      event "Delayed Interlace Start": Value Change {
        n1232 = event-data() -> ()  [unwired: 7 out]
        n1233 = flat-sequence {
          frame #0 {
            n1234 = Multiply(x="Delay to Interlace (s)", y=1000.0) -> (x*y=w1976:dbl)
            n1235 = Wait (ms)(milliseconds to wait=w1976) -> ()  [unwired: 1 out]
          }
          frame #1 {
            n1236 = property on="Laser interlacing mode" class="RadioBtnsControl (strict)"("Val(Sgnl)"=enum32{"Laser ON", "Laser OFF", "Interlace"}."Interlace" ("Value (Signaling)")) -> ()  [unwired: 2 in, 2 out]
          }
        }
      }
      event "BD 1 Amplitude 1 (%)", "BD 1 Amplitude 2 (%)", "BD 1 Amplitude 3 (%)", "BD 2 Amplitude 1 (%)", "BD 2 Amplitude 2 (%)", "BD 2 Amplitude 3 (%)", "Trap 1 ON", "Trap 2 ON", "Trap 3 ON", "Feedback On/Off", "All FB On/Off": Value Change {
        w2001 = i16 1 ("f")
        n1237 = event-data() -> ()  [unwired: 7 out]
        n1238 = local write "Trap 1 (ON/OFF)"("Trap 1 ON") -> ()
        n1239 = local write "Trap 2 (ON/OFF)"("Trap 2 ON") -> ()
        n1240 = Boolean To (0,1)(Boolean="Trap 3 ON") -> (0, 1=w2002:i16)
        n1241 = Boolean To (0,1)(Boolean="Trap 1 ON") -> (0, 1=w2003:i16)
        n1242 = Boolean To (0,1)(Boolean="Trap 2 ON") -> (0, 1=w2004:i16)
        n1243 = Select(t=w2004, s="Trap ON/OFF X or Y Amp?", f=w2001) -> (s? t:f=w1999:i16)
        n1244 = Select(t=w2003, s="Trap ON/OFF X or Y Amp?", f=w2001) -> (s? t:f=w2000:i16)
        n1245 = Select(t=w2002, s="Trap ON/OFF X or Y Amp?", f=w2001) -> (s? t:f=w1998:i16)
        n1246 = Select(t=w2001, s="Trap ON/OFF X or Y Amp?", f=w2004) -> (s? t:f=w1996:i16)
        n1247 = Select(t=w2001, s="Trap ON/OFF X or Y Amp?", f=w2003) -> (s? t:f=w1997:i16)
        n1248 = Select(t=w2001, s="Trap ON/OFF X or Y Amp?", f=w2002) -> (s? t:f=w1995:i16)
        n1249 = And(x="All FB On/Off", y="Feedback On/Off") -> (x .and. y?=w1993:cluster{"Set 1":bool, "Set 2":bool})
        n1250 = local read "BD 1 Amplitude 1 (%)"() -> (w2011:dbl)
        n1251 = local read "BD 1 Amplitude 2 (%)"() -> (w2010:dbl)
        n1252 = local read "BD 1 Amplitude 3 (%)"() -> (w2009:dbl)
        n1253 = Unbundle By Name(w1993) -> ("Set 1"=w1988:bool, "Set 2"=w1985:bool)
        n1254 = local read "Y RF Amplitude Limits (%)"() -> (w1981:T26)
        n1255 = local read "X RF Amplitude Limits (%)"() -> (w1982:T26)
        n1256 = local read "BD 2 Amplitude 1 (%)"() -> (w2012:dbl)
        n1257 = local read "BD 2 Amplitude 2 (%)"() -> (w2013:dbl)
        n1258 = local read "BD 2 Amplitude 3 (%)"() -> (w2014:dbl)
        n1259 = And(x="Trap 2 ON", y=w1985) -> (x .and. y?=w1983:bool)
        n1260 = And(x="Trap 1 ON", y=w1988) -> (x .and. y?=w1986:bool)
        n1261 = Multiply(x=w2000, y=w2011) -> (x*y=w2008:dbl)
        n1262 = Multiply(x=w2010, y=w1999) -> (x*y=w2006:dbl)
        n1263 = Multiply(x=w2009, y=w1998) -> (x*y=w2007:dbl)
        n1264 = Multiply(x=w2012, y=w1997) -> (x*y=w2015:dbl)
        n1265 = Multiply(x=w2013, y=w1996) -> (x*y=w2016:dbl)
        n1266 = Multiply(x=w2014, y=w1995) -> (x*y=w2017:dbl)
        n1267 = call "set RF board amplitude - interlace.vi"("Board 2 Amplitude Limits"=w1981, "Board 1 Amplitude Limits"=w1982, "FPGA VI Reference In"=w1980, "Board 2 Amplitude 3 (%)"=w2017, "Board 1 Amplitude 3 (%)"=w2007, "Board 2 Amplitude 2 (%)"=w2016, "Board 2 Amplitude 1 (%)"=w2015, "Board 1 Amplitude 2 (%)"=w2006, "Board 1 Amplitude 1 (%)"=w2008) -> ("error out"=w1990:errorcluster, "FPGA VI Reference Out"=w1991:T40)  [unwired: 1 in]
        n1268 = xnode "Read/Write Control"("FPGA VI Reference In"=w1991, "error in"=w1990, "FB On/Off Set 1"=w1986, "FB On/Off Set 2"=w1983) -> ("error out"=w1989:errorcluster)  [unwired: 1 out]
      }
      event "Load parameters": Value Change {
        n1269 = event-data() -> ()  [unwired: 7 out]
        n1270 = property on="Saved AOD Raster Scan Parameter Sets" class="Arr (strict)"() -> ("Index Values"=w2028:u32[])  [unwired: 2 in, 2 out]
        n1271 = Index Array(array=w2028, index=0) -> (element=w2025:u32)
        n1272 = local write "Load parameters"(FALSE ("Load parameters")) -> ()
        n1273 = Index Array(array="Saved AOD Raster Scan Parameter Sets", index=w2025) -> (element=w2024:T54)
        n1274 = Unbundle By Name(w2024) -> ("Scan Range AOD (nm) 2"=w2023:dbl, "Step Size AOD (nm) 2"=w2022:dbl, "Scan Speed AOD (nm/s) 2"=w2021:dbl, "Number of scans (AOD) 2"=w2020:u16)
        n1275 = flat-sequence {
          tunnel: w2023 -> [w2031]
          tunnel: w2022 -> [w2030]
          tunnel: w2021 -> [w2029]
          tunnel: w2020 -> [w2032]
          frame #0 {
            n1276 = local write "Scan Speed (nm/s)"(w2029) -> ()
            n1277 = local write "Scan Range (nm)"(w2031) -> ()
            n1278 = local write "Step Size (nm)"(w2030) -> ()
          }
          frame #1 {
            n1279 = property on="Number of F/B Scans (AOD)" class="DigNum (strict)"("Val(Sgnl)"=w2032) -> ()  [unwired: 2 in, 2 out]
          }
        }
      }
      event "Trap 1 (ON/OFF)", "Trap 2 (ON/OFF)": Value Change {
        n1280 = event-data() -> ()  [unwired: 7 out]
        n1281 = flat-sequence {
          tunnel: [w2042] -> w2037
          tunnel: w2037 -> [w2057]
          tunnel: [w2043] -> w2033
          frame #0 {
            n1282 = local read "Trap 1 ON"() -> (w2042:bool)
          }
          frame #1 {
            n1283 = Exclusive Or(1:w2057, 2:"Trap 1 (ON/OFF)") -> (0:w2050:bool)
            n1284 = Select(t="on", s="Trap 2 (ON/OFF)", f="off") -> (s? t:f=w2049:string)
            n1285 = Select(t="on", s="Trap 1 (ON/OFF)", f="off") -> (s? t:f=w2045:string)
            n1286 = Build Array("trap 1 ", w2045) -> (w2044:string[])
            n1287 = Build Array("trap 2 " ("f"), w2049) -> (w2047:string[])
            n1288 = Select(t=w2044, s=w2050, f=w2047) -> (s? t:f=w2043:string[])
            n1289 = property on="Trap 1 ON" class="Bool (strict)"("Val(Sgnl)"="Trap 1 (ON/OFF)") -> ()  [unwired: 2 in, 2 out]
            n1290 = property on="Trap 2 ON" class="Bool (strict)"("Val(Sgnl)"="Trap 2 (ON/OFF)") -> ()  [unwired: 2 in, 2 out]
          }
        }
        n1291 = local read "Saving..."() -> (w2036:bool)
        n1292 = local read "Save Event Log?"() -> (w2035:bool)
        n1293 = And(x=w2036, y=w2035) -> (x .and. y?=w2034:bool)
        n1294 = case shown="True" w2034 {
          tunnel: w2033 -> [_ w2041]
          frame False {
          }
          frame True {
            n1295 = local read "Time (s)"() -> (w2038:dbl)
            n1296 = local read "log file ref"() -> (w2040:refnum<file>)
            n1297 = Concatenate Strings(w2041) -> (w2039:string)
            n1298 = call "write to event log.vi"("log file ref"=w2040, "time"=w2038, "input string"=w2039) -> ()  [unwired: 8 in]
          }
        }
      }
      event "DIO count 1 (ticks)", "DIO count 2 (ticks)", "DIO count 3 (ticks)", "Interlace", "Number Interlace Sets", "Not-Interlacing Set", "BD 1 Delay (ticks)", "BD 2 Delay (Ticks)", "Next trap write delay (ticks)", "Phase offset method", "Phase Increment Trap 1", "Phase Increment Trap 2", "RF phase reset before cycles": Value Change {
        n1299 = event-data() -> ()  [unwired: 7 out]
        n1300 = To Unsigned Byte Integer(number="Not-Interlacing Set") -> (unsigned 8bit integer=w2062:u8)
        n1301 = Add(x=u8 1 ("y"), y=w2062) -> (x+y=w2071:u8)
        n1302 = local read "DIO count 1 (ticks)"() -> (w2078:u16)
        n1303 = local read "DIO count 2 (ticks)"() -> (w2077:u16)
        n1304 = local read "DIO count 3 (ticks)"() -> (w2076:u16)
        n1305 = local read "RF phase reset before cycles"() -> (w2058:bool)
        n1306 = local read "Phase Increment Trap 1"() -> (w2060:fxp<+,14,14>)
        n1307 = local read "Phase offset method"() -> (w2061:u8)
        n1308 = local read "Phase Increment Trap 2"() -> (w2059:fxp<+,14,14>)
        n1309 = xnode "Read/Write Control"("FPGA VI Reference In"=w2064, "DIO count 1 (ticks)"=w2078, "DIO count 2 (ticks)"=w2077, "DIO count 3 (ticks)"=w2076, "Interlace ON/OFF"="Interlace", "Number Interlace Cycles"="Number Interlace Sets", "Interlace Off Parameters"=w2071, "BD 1 Delay (ticks)"="BD 1 Delay (ticks)", "BD 2 Delay (Ticks)"="BD 2 Delay (Ticks)", "Next trap write delay (ticks)"="Next trap write delay (ticks)", "Phase offset method"=w2061, "Phase Trap 1"=w2060, "Phase Trap 2"=w2059, "RF phase reset before cycles"=w2058) -> ("error out"=w2080:errorcluster)  [unwired: 1 in, 1 out]
        n1310 = Build Array(w2078, w2077, w2076) -> (w2070:u16[])
        n1311 = Split 1D Array(array=w2070, index="Number Interlace Sets") -> (first subarray=w2079:u16[])  [unwired: 1 out]
        n1312 = Index Array(array=w2070, index=w2062) -> (element=w2069:u16)
        n1313 = Add Array Elements(numeric array=w2079) -> (sum=w2073:u16)
        n1314 = Select(t=w2073, s="Interlace", f=w2069) -> (s? t:f=→"Total Counts (ticks)":u16)
      }
      event "Reset Feedback": Value Change {
        n1315 = event-data() -> ()  [unwired: 7 out]
        n1316 = Unbundle By Name("Reset Feedback") -> ("Set 1"=w2084:bool, "Set 2"=w2083:bool)
        n1317 = xnode "Read/Write Control"("FPGA VI Reference In"=w2081, "FB Reset Set 1"=w2084, "FB Reset Set 2"=w2083) -> ("error out"=w2082:errorcluster)  [unwired: 1 in, 1 out]
      }
      event "Trap intensity output range", "Trap Intensity PID Gains": Value Change {
        n1318 = event-data() -> ()  [unwired: 7 out]
        n1319 = xnode "Read/Write Control"("FPGA VI Reference In"=w2088, "FB Gains"="Trap Intensity PID Gains", "FB output range"="Trap intensity output range") -> ("error out"=w2089:errorcluster)  [unwired: 1 in, 1 out]
      }
      event "AI2 to Setpoint", "Setpoints (V)": Value Change {
        n1320 = event-data() -> ()  [unwired: 7 out]
        n1321 = xnode "Read/Write Control"("FPGA VI Reference In"=w2090) -> ("FPGA VI Reference Out"=w2093:T40, "error out"=w2092:errorcluster, "AI2 Y Sum Set 1"=w2100:i16, "AI2 Y Sum Set 2"=w2099:i16)  [unwired: 1 in]
        n1322 = Cluster To Array(cluster="AI2 to Setpoint") -> (array=w2103:bool[])
        n1323 = local read "AI2 (V)"() -> (w2101:cluster{"Set 1":dbl, "Set 2":dbl})
        n1324 = Or Array Elements(Boolean array=w2103) -> (logical OR=w2104:bool)
        n1325 = Bundle By Name(cluster=w2101, "Set 1"=w2100, "Set 2"=w2099) -> (w2098:cluster{"Set 1":dbl, "Set 2":dbl})
        n1326 = Divide(x=w2098, y=3276.7) -> (x/y=w2097:cluster{"Set 1":dbl, "Set 2":dbl})
        "AI2 (V)" <- w2097
        n1327 = case shown="True" w2104 {
          tunnel: [w2107 w2124] -> w2096
          tunnel: "AI2 to Setpoint" -> [_ w2120]
          tunnel: "Setpoints (V)" -> [w2108 w2123]
          tunnel: w2097 -> [_ w2117]
          frame False {
            n1328 = Multiply(x=3276.7, y=w2108) -> (x*y=w2109:cluster{"Set 1":dbl, "Set 2":dbl})
            n1329 = To Word Integer(number=w2109) -> (16bit integer=w2107:cluster{"Set 1":i16, "Set 2":i16})
          }
          frame True {
            n1330 = Unbundle By Name(w2117) -> ("Set 1"=w2116:dbl, "Set 2"=w2115:dbl)
            n1331 = Unbundle By Name(w2123) -> ("Set 1"=w2122:dbl, "Set 2"=w2121:dbl)
            n1332 = Unbundle By Name(w2120) -> ("Set 1"=w2119:bool, "Set 2"=w2118:bool)
            n1333 = Select(t=w2116, s=w2119, f=w2122) -> (s? t:f=w2114:dbl)
            n1334 = Select(t=w2115, s=w2118, f=w2121) -> (s? t:f=w2113:dbl)
            n1335 = Bundle By Name(cluster=w2123, "Set 1"=w2114, "Set 2"=w2113) -> (w2111:cluster{"Set 1":dbl, "Set 2":dbl})
            n1336 = local write "Setpoints (V)"(w2111) -> ()
            n1337 = Multiply(x=3276.7, y=w2111) -> (x*y=w2112:cluster{"Set 1":dbl, "Set 2":dbl})
            n1338 = To Word Integer(number=w2112) -> (16bit integer=w2124:cluster{"Set 1":i16, "Set 2":i16})
          }
        }
        n1339 = Unbundle By Name(w2096) -> ("Set 1"=w2095:i16, "Set 2"=w2094:i16)
        n1340 = xnode "Read/Write Control"("FPGA VI Reference In"=w2093, "error in"=w2092, "FB Setpoint Set 1"=w2095, "FB Setpoint Set 2"=w2094) -> ("error out"=w2091:errorcluster)  [unwired: 1 out]
      }
      event "+ phase (GI)", "- phase (GI)", "+ phase (GI) 2", "- phase (GI) 2", "+ phase (RI)", "- phase (RI)", "+ phase (Green FB)", "- phase (Green FB)", "- phase (BI AO)", "+ phase (BI AO)", "- phase (BI DO)", "+ phase (BI DO)": Value Change {
        n1341 = event-data() -> ()  [unwired: 7 out]
        n1342 = Or(x="+ phase (GI)", y="- phase (GI)") -> (x .or. y?=w2160:bool)
        n1343 = Negate(x="Phase adj. (GI)") -> (-x=w2165:i16)
        n1344 = Select(t=w2165, s="+ phase (GI)", f="Phase adj. (GI)") -> (s? t:f=w2164:i16)
        n1345 = Or(x="+ phase (GI) 2", y="- phase (GI) 2") -> (x .or. y?=w2151:bool)
        n1346 = Negate(x="Phase adj. (GI) 2") -> (-x=w2156:i16)
        n1347 = Select(t=w2156, s="+ phase (GI) 2", f="Phase adj. (GI) 2") -> (s? t:f=w2152:i16)
        n1348 = Negate(x="Phase adj. (RI)") -> (-x=w2150:i16)
        n1349 = Or(x="+ phase (RI)", y="- phase (RI)") -> (x .or. y?=w2146:bool)
        n1350 = Select(t=w2150, s="+ phase (RI)", f="Phase adj. (RI)") -> (s? t:f=w2145:i16)
        n1351 = Or(x="+ phase (Green FB)", y="- phase (Green FB)") -> (x .or. y?=w2139:bool)
        n1352 = Negate(x="Phase adj. (Green FB)") -> (-x=w2144:i16)
        n1353 = Select(t=w2144, s="+ phase (Green FB)", f="Phase adj. (Green FB)") -> (s? t:f=w2140:i16)
        n1354 = Negate(x="Phase adj. (BI AO)") -> (-x=w2138:i16)
        n1355 = Or(x="+ phase (BI AO)", y="- phase (BI AO)") -> (x .or. y?=w2128:bool)
        n1356 = Select(t=w2138, s="+ phase (BI AO)", f="Phase adj. (BI AO)") -> (s? t:f=w2130:i16)
        n1357 = Negate(x="Phase adj. (BI DO)") -> (-x=w2134:i16)
        n1358 = Or(x="+ phase (BI DO)", y="- phase (BI DO)") -> (x .or. y?=w2127:bool)
        n1359 = Select(t=w2134, s="+ phase (BI DO)", f="Phase adj. (BI DO)") -> (s? t:f=w2129:i16)
        n1360 = xnode "Read/Write Control"("FPGA VI Reference In"=w2126, "Phase count adjustment (GI)"=w2164, "Phase count adjustment (GI) 2"=w2152, "Phase count adjustment (RI)"=w2145, "Phase count adjustment (Green FB)"=w2140, "Phase count adjustment (BI AO)"=w2130, "Phase count adjustment (BI D)"=w2129) -> ("FPGA VI Reference Out"=w2162:T40, "error out"=w2163:errorcluster)  [unwired: 1 in]
        n1361 = xnode "Read/Write Control"("FPGA VI Reference In"=w2162, "error in"=w2163, "+ phase (GI)"=w2160, "+ phase (GI) 2"=w2151, "+ phase (RI)"=w2146, "+ phase (Green FB)"=w2139, "+ phase (BI AO)"=w2128, "+ phase (BI D)"=w2127) -> ("error out"=w2161:errorcluster)  [unwired: 1 out]
      }
      event "Green Laser ON/OFF", "Red Laser ON/OFF", "Blue Laser ON/OFF": Value Change {
        # "This loop shouldn't be initialized.  The main 'laser ON' settings should dominate and set the others."
        n1362 = event-data() -> ()  [unwired: 7 out]
        n1363 = property on="Red Laser ON" class="Bool (strict)"("Val(Sgnl)"="Red Laser ON/OFF") -> ()  [unwired: 2 in, 2 out]
        n1364 = property on="Blue Laser ON" class="Bool (strict)"("Val(Sgnl)"="Blue Laser ON/OFF") -> ()  [unwired: 2 in, 2 out]
        n1365 = property on="Green Laser ON" class="Bool (strict)"("Val(Sgnl)"="Green Laser ON/OFF") -> ()  [unwired: 2 in, 2 out]
      }
      event "Laser interlacing mode", "Green Laser ON", "Red Laser ON", "Blue Laser ON": Value Change {
        n1366 = event-data() -> ()  [unwired: 7 out]
        n1367 = local write "Green Laser ON/OFF"("Green Laser ON") -> ()
        n1368 = local write "Blue Laser ON/OFF"("Blue Laser ON") -> ()
        n1369 = local write "Red Laser ON/OFF"("Red Laser ON") -> ()
        n1370 = case shown="False" "Green Laser ON" {
          tunnel: "Laser interlacing mode" -> [_ w2226]
          tunnel: [enum32{"Laser ON", "Laser OFF", "Interlace"}."Laser OFF" ("Green laser mode") w2226] -> w2202